vi "test_lut.vi"(6 "Use range":sgl[](array[numeric])=[0.8, 0.8, 0.8, 0.15], 8 "Random probes":i32=400000, 9 "Calibration data":T3, 10 "LUT":T2={"Table"=array41x41x41x5x4[1378420 elements], "Scale"=[2.0, 2.0, 2.0, 0.11], "Offset"=[-1.0, -1.0, -1.0, -0.03]}) -> (2 "Results":T1 {"Max error axis positions" format="%#.4f"; "RMS error" format="%#.1f"; "Max error" format="%#.1f"})   [LabVIEW 2012]
uses:
  initialization/asap_calibration.ctl
  <vilib>/Analysis/Matrix/Datatypes/RealMatrix.ctl
  geometry/lut4d.ctl
  <vilib>/Analysis/Matrix/NI_Matrix.lvlib
panel:
  # "Test over +/- this range of normalized values.   There are boundary conditions at the edges of the LUT, and the entire sensor doesn't give usable data anyway."
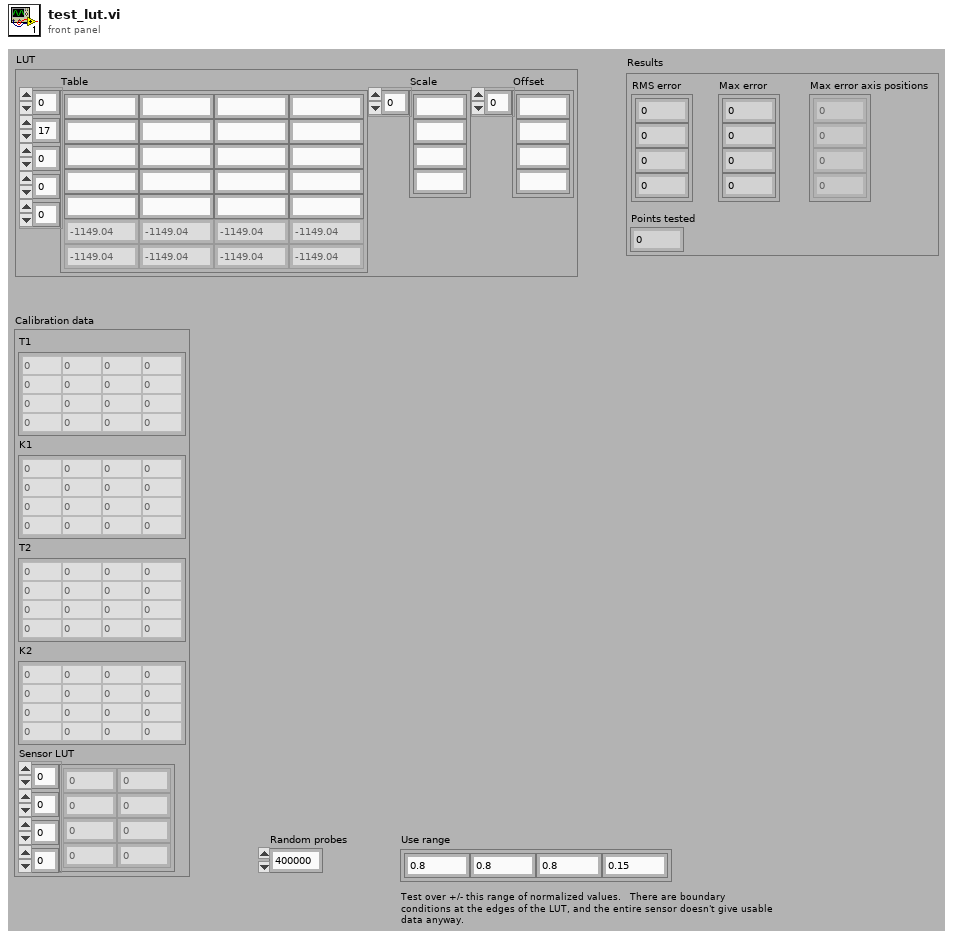
[diagram p1: front panel]
types:
  T1 = cluster{"Max error":sgl[], "Points tested":i32, "RMS error":sgl[], "Max error axis positions":sgl[]}
  T2 = typedef "lut4d.ctl" = cluster{"Table":sgl[][][][][], "Scale":sgl[], "Offset":sgl[]}
  T3 = typedef "asap_calibration.ctl" = cluster{"T1":T4, "K1":T4, "T2":T4, "K2":T4, "Sensor LUT":sgl[][][][]}
  T4 = typedef "NI_Matrix.lvlib/RealMatrix.ctl" = dbl[][]
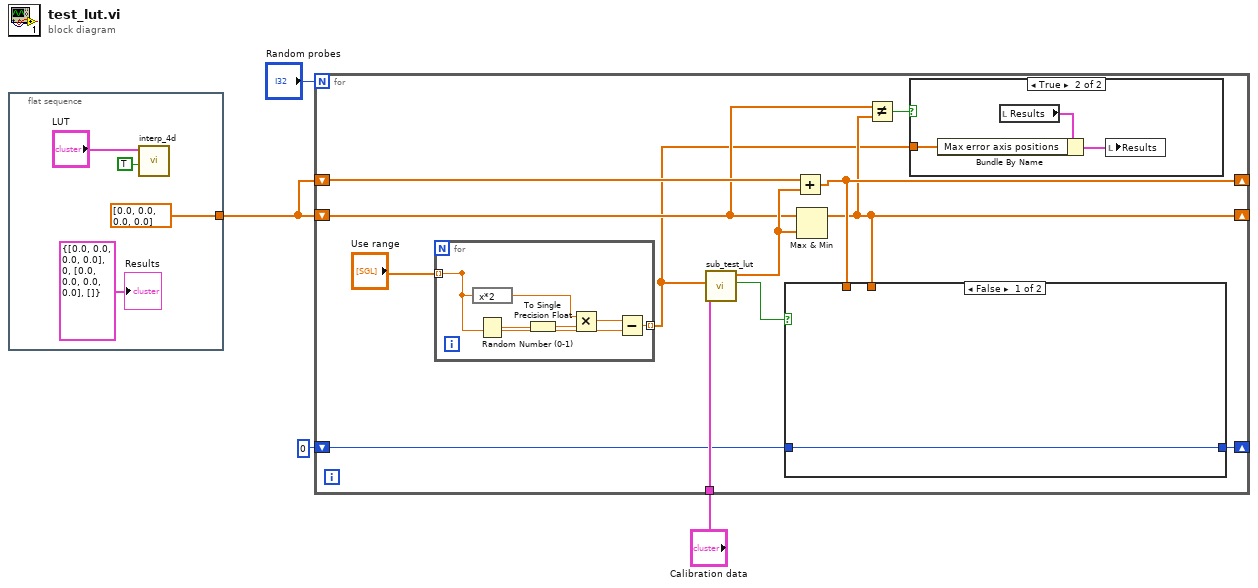
[diagram p0: block diagram]
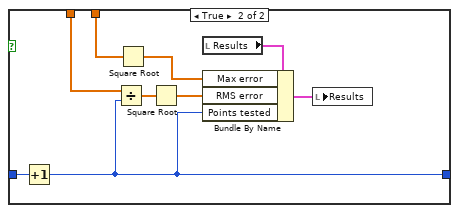
[diagram p3: hidden frame]
diagram:
  n1 = flat-sequence {
    tunnel: [sgl[] [0.0, 0.0, 0.0, 0.0] ("Array 2")] -> w2
    frame #0 {
      n2 = call "interp_4d.vi"("Set LUT"=TRUE, "LUT"="LUT") -> ()  [unwired: 9 in, 1 out]
      "Results" <- T1 {"Max error"=[0.0, 0.0, 0.0, 0.0], "Points tested"=0, "RMS error"=[0.0, 0.0, 0.0, 0.0], "Max error axis positions"=[]} ("Results")
    }
  }
  n3 = for {
    N: "Random probes" -> [_]
    tunnel: "Calibration data" -> [w19]
    shift-right: [w13] -> _
    shift-left: w2 -> [w14]
    shift-right: [w16] -> _
    shift-left: w2 -> [w17]
    shift-right: [w9] -> _
    shift-left: 0 ("Points tested") -> [w10]
    n4 = for {
      tunnel: [w35] -> _ mode=indexing
      tunnel: "Use range" -> [w35] mode=indexing
      tunnel: [w34] -> w11 mode=indexing
      n5 = expression code="x*2"(w35) -> (w39:sgl)
      n6 = Random Number (0-1)() -> (number: 0 to 1=w38:dbl)
      n7 = To Single Precision Float(number=w38) -> (single precision float=w37:sgl)
      n8 = Multiply(x=w39, y=w37) -> (x*y=w36:sgl)
      n9 = Subtract(x=w36, y=w35) -> (x-y=w34:sgl)
    }
    n10 = call "sub_test_lut.vi"("Calibration data"=w19, "Normalized axis positions"=w11) -> ("Plausible point"=w20:bool, "Error squared"=w18:sgl[])  [unwired: 8 in]
    n11 = Add(x=w17, y=w18) -> (x+y=w16:sgl[])
    n12 = Max & Min(x=w14, y=w18) -> (max(x,y)=w13:sgl[])  [unwired: 1 out]
    n13 = case shown="False" w20 {
      tunnel: w13 -> [_ w33]
      tunnel: w16 -> [_ w32]
      tunnel: w10 -> [w24 w30]
      tunnel: [w24 w26] -> w9
      frame False {
      }
      frame True {
        n14 = Increment(x=w30) -> (x+1=w26:i32)
        n15 = Divide(x=w32, y=w26) -> (x/y=w31:sgl[])
        n16 = Square Root(x=w33) -> (sqrt(x)=w28:sgl[])
        n17 = Square Root(x=w31) -> (sqrt(x)=w27:sgl[])
        n18 = local read "Results"() -> (w29:T1)
        n19 = Bundle By Name(cluster=w29, "Max error"=w28, "RMS error"=w27, "Points tested"=w26) -> (w25:T1)
        n20 = local write "Results"(w25) -> ()
      }
    }
    n21 = Not Equal?(x=w14, y=w13) -> (x != y?=w12:bool)
    n22 = case shown="True" w12 {
      tunnel: w11 -> [_ w21]
      frame False {
      }
      frame True {
        n23 = local read "Results"() -> (w22:T1)
        n24 = Bundle By Name(cluster=w22, "Max error axis positions"=w21) -> (w23:T1)
        n25 = local write "Results"(w23) -> ()
      }
    }
  }
